vi "UHR-Fleezers Control (host) - Avogadro v2.vi"() -> ()   [LabVIEW 2014]
uses:
  <vilib>/Utility/miscctls.llb/LVPoint32TypeDef.ctl
  <vilib>/Utility/miscctls.llb/LVMinMaxIncTypeDef.ctl
  <vilib>/addons/database/Connection.llb/Conn ObjectReference.ctl
  <vilib>/sound2/lvsound2.llb/Sampling Mode.ctl
  <vilib>/sound2/lvsound2.llb/Sound Data Format.ctl
  <vilib>/Platform/TimedLoop/XDataNode/timing_clust.ctl
  <vilib>/Platform/TimedLoop/XDataNode/nitl_modes.ctl
  <vilib>/Platform/TimedLoop/XDataNode/wakeup.ctl
  uFLUX control_v2/uFLUX control_v2/Pressure Control/Pressure Control.lvclass
  uFLUX control_v2/uFLUX control_v2/TTL/TTL.lvclass
  uFLUX control_v2/uFLUX control_v2/Pressure Control/Pressure Control Config.ctl
  <vilib>/userdefined/High Color/nirio_resource_hc.ctl
  <vilib>/Analysis/baseanly.llb/Mean (DBL).vi
  <vilib>/Instr/_visa.llb/VISA Configure Serial Port (Instr).vi
  <vilib>/FPGAPlugInAG/PCIe-7852R/niLvFpga_Open_PCIe-7852R.vi
  <vilib>/FPGAPlugInAG/PCIe-7852R/niLvFpga_Reset_PCIe-7852R.vi
  <vilib>/FPGAPlugInAG/PCIe-7852R/niLvFpga_Run_PCIe-7852R.vi
  <vilib>/FPGAPlugInAG/PCIe-7852R/niLvFpga_Close_PCIe-7852R.vi
  <vilib>/Utility/error.llb/Error Cluster From Error Code.vi
  <vilib>/rvi/errors/niLvFpgaAdjustHostInterfaceError.vi
  <vilib>/rvi/interface/common/niFpgaWaitOnOcc.vi
  <vilib>/express/express analysis/Spectral/Block/exnSpectralBlock spectral measurements PSD poly.vi
  <vilib>/express/express analysis/Spectral/Block/exnSpectralBlock spectral measurements PSD WFM.vi
  <vilib>/Waveform/WDTOps.llb/WDT Append Waveforms DBL.vi
  <vilib>/Waveform/WDTOps.llb/WDT Index Channel DBL.vi
  <vilib>/sound2/lvsound2.llb/Sound Output Write (DBL Single).vi
  openfpgaref.8.6.ctl
  <vilib>/Platform/TimedLoop/XDataNode/XDataNode.xnode
  <vilib>/rvi/interface/nirviOpenFPGA/nirviOpenFPGA.xnode
  openfpgaref.initrf.ctl
  FPGA Bitfiles/UHR-FleezersInst_FPGATarget_intitializeRFsyn_v1.lvbitx
  <vilib>/rvi/interface/nirviMethod/nirviMethod.xnode
  <vilib>/rvi/interface/nirviCloseFPGA/nirviCloseFPGA.xnode
  FPGA Bitfiles/UHR-FleezersInst_FPGATarget_UHR-FleezersCont_avogadro4_switch_test.lvbitx
  <vilib>/rvi/interface/nirviReadWriteControl/nirviReadWriteControl.xnode
  <vilib>/express/express analysis/Spectral/XNode/ExpressSpectralMeasurementsBlockNode.xnode
  <vilib>/Analysis/NI_AALBase.lvlib
  <vilib>/Platform/TimedLoop/XDataNode/XDNodeRunTimeDep.lvlib
  Duncan Nall/Fluorescence simulation/Global for fluorescence simulation mean (30 samples), (power series).vi
  <vilib>/gmath/NI_Gmath.lvlib
  <vilib>/addons/database/NI_Database_API.lvlib
  <vilib>/rvi/errors/niLvFpgaMergeErrorWithErrorCode.vi
  NiFpgaLv.dll
  <vilib>/FPGAPlugInAG/PCIe-7852R/niLvFpga_ConfigureFifo_PCIe-7852R.vi
  <vilib>/FPGAPlugInAG/PCIe-7852R/niLvFpga_ReadFifo_PCIe-7852R.vi
  <vilib>/addons/database/Connection.llb/DB Tools Open Connec (Path).vi
panel:
  out "2D values (force/position/raw)":T1={"A_X"=10.819281125703213, "A_Y"=-5.499317852510465, "B_X"=12.368914072758173, "B_Y"=-10.556033598869238, "C_X"=11.443452130367886, "C_Y"=-14.04467976971868}
  out "APD rates cluster":T2={"APD 1 Rate (Hz)"=4.0, "APD 2 Rate (Hz)"=0.0, "APD 3 Rate (Hz)"=0.0, "Sigma/Mean 1"=nan, "Int Time (s)"=4.0, "Sigma 1"=0.0, "Sigma 2"=0.0, "Sigma 3"=0.0, "Sigma/Mean 2"=nan, "Sigma/Mean 3"=nan}
  out "Read offset current":string(combo)
  out "PSD Y Sum":dbl[](array[numeric])
  out "log file ref":refnum<file>
  out "AL Running":bool
  in  "AL Delay (s)":u32
  in  "Stop assembly line":bool
  in  "Cy5 Fl.  Thresh. (kHz)":dbl=24.5
  in  "Cy3 Fl.  Thresh. (kHz)":dbl=19.0
  in  "Get Fluorophore":bool
  out "Red Fluorophore":bool
  out "Green Fluorophore":bool
  in  "Numeric":dbl
  in  "stop":bool
  in  "Start assembly line":bool
  out "HP3 Flush Time (s)":dbl=90.0
  out "HP1 Flush Time (s)":dbl=60.0
  out "TTrig":cluster{dbl, dbl}(graph)
  in  "Sample Channel\nFlow":bool
  in  "Inject Pump 1":bool
  in  "Inject Pump 3":bool
  in  "Pump 1 contents":string="Bottom: DNA beads" caption="Contents"
  in  "Pump 3 contents":string="Top: ADig beads" caption="Contents"
  in  "Scripts":T3(tab)=enum."Saving"
  in  "Experiment position":bool
  in  "Get Bead 1":bool
  in  "Fixed Traps Data\nScript":bool
  in  "Dump spot flow on?":bool=TRUE caption="Flow ON?"
  in  "Daq spot flow on":bool=TRUE caption="Flow ON?"
  in  "Cap 1 Samp Flow ON":bool=TRUE
  in  "Cap 2 Samp Flow ON":bool=TRUE
  in  "Get bead 2":bool
  in  "Get bead 3":bool
  in  "Cap 2 Flow ON":bool=TRUE
  in  "Cap 1 Flow ON":bool=TRUE
  in  "Cap 2 T ON":bool=TRUE
  in  "Move Cap. 2 (ADig Top)":bool
  in  "Move Cap. 1 (DNA Bottom)":bool
  in  "Cal/Data Acq. Spot":bool
  in  "Dump Beads":bool
  in  "Cap 1 T ON":bool=TRUE
  in  "Force FB Data\nScript":bool
  in  "Cap. 2 BD T1?\n(ADig T1, DNA T2)":bool
  in  "Flow Cal":bool
  in  "Pulse Duration (0-100 ms)":dbl=10.0
  in  "Number of pulses For laminar flow":i32=1
  in  "Vent pressure":bool
  in  "Pressure Up":bool=TRUE
  in  "Pressure Down":bool=TRUE
  out "Pressure":dbl=0.010543157373989365 format="%#.2f"
  in  "Set zero pressure":bool caption="Vent pressure"
  in  "Vacuum":bool=TRUE
  in  "DAQmx Device Name":tag="Dev1"
  in  "Offset raster?":bool
  in  "MCL offset scanning range (V)":T4={"Min X"=6.0, "Max X"=9.0, "Min Y"=5.0, "Max Y"=8.0, "Scan increment"=1.0}
  in  "Multiple-MCL offset?":bool=TRUE
  in  "Active cal after cal?":bool
  in  "Fish after cal?":bool
  in  "Flow ON during cal?":bool
  in  "Offset 2 Set":dbl=3.0
  in  "Offset 1 Set":dbl
  in  "Cal @ (MHz)":dbl=14.0
  in  "W/ Offset 1":bool
  in  "Offset 1 Start (MHz)":dbl=10.0
  in  "W/ Offset 2":bool
  in  "Offset 2 Start (MHz)":dbl=10.0
  in  "Cal Stage Position":i32=3
  in  "Index":dbl=1.0 caption="Save File Index" min=1.0 step=1.0
  out "Time (s)":dbl=12.200000000000001
  in  "Channel 3 Buffer":string="NA"
  in  "Channel 2 Buffer":string="NA"
  out "Save Data Period (s)":dbl=0.001 caption="Period (s)" format="%#_6p"
  out "Save Data Rate (Hz)":dbl=1000.0 caption="Rate (Hz)" format="%#_6p"
  out "Progress":u16(slide) scale=0.0..100.0
  in  "Stop Saving":bool
  out "Saving...":bool
  in  "Save ave N":dbl=100.0 caption="Averaging Factor"
  out "Save file name":path=path "C:/Data/180326/180326_017.dat"
  in  "Save N Sets":bool
  in  "N sets to save":u32=200 caption="N Sets"
  out "Calibrating Trap...":bool
  in  "Comment (data description)":string="testing confocal setup"
  in  "Start Saving":bool
  out "Total Time (s) 2":dbl=40.0
  in  "Name":string="test name"
  in  "Title":string="testing database"
  in  "DNA Construct":string="oligo binding"
  in  "Channel 1 Buffer":string
  in  "Bead diameter":dbl=800.0
  in  "Save Event Log?":bool=TRUE
  in  "Only check fixed trap T2":bool
  in  "Flow ON after\ntether testing?":bool
  in  "Flow ON during \nfishing?":bool
  in  "Fish again after \nraster break?":bool
  in  "Furthest Delta (MHz)":dbl=15.0 step=0.25
  in  "Green ON During Raster":bool
  in  "Move to Delta 2 (MHz)":dbl=12.3
  in  "Attempt Limit":dbl=20.0 caption="Limit"
  out "Attempts":dbl=10.0
  in  "Wait Before Save (s)":u32=1
  in  "Closest Delta (MHz)":dbl=8.0 step=0.25
  in  "Stop F (pN)":dbl=3.0
  in  "Then...":string(combo)="5"
  in  "Move to Delta 1 (MHz)":dbl=10.0
  in  "Tether Alarm?":bool=TRUE
  out "Tether":bool
  in  "TA Cancel Save?":bool
  in  "TA Green Off?":bool
  in  "Raster Set Upon Tether":u32=5
  in  "Save at end (5, 6)":bool
  in  "Stop Fishing When Tether":bool=TRUE
  in  "Delay before dipping (s)":dbl=5.0
  in  "Start dipping after?":bool
  in  "Green ON after FB ON?":bool
  in  "Remove Action Offset":bool
  in  "Stage Position To Establish FB":i32=3
  in  "Trap Trig Fl.":bool
  in  "Starting \nTrap Delta (MHz)":dbl=15.25
  in  "Trap Delta Before Moving":dbl=13.0
  in  "Wait (s)":u32=1
  in  "Green ON":bool
  in  "Start dipping after?":bool=TRUE
  in  "Fixed Traps Trap Delta (MHz)":dbl=15.25 caption="Trap Delta (MHz)"
  out "TTrig Fin Thresh (nm)":dbl
  out "TTrig Sig (nm)":dbl
  out "Threshold stored (nm)":dbl
  in  "Neg. TTrig FPGA":bool=TRUE
  in  "Test ttrig":bool
  in  "Trap Trig. (FPGA)":bool=TRUE
  out "Initializing":bool
  in  "Reinitialize":bool
  out "Triggered":bool
  out "Waiting":bool
  in  "Trap Trig. Fl.":bool
  in  "Wait to get offset (n)":u32=10
  in  "Threshold (nm)":dbl=15.0
  in  "Fl. ON time (n)":i32=90
  out "max value":dbl=-0.9003514563721442
  out "min value":dbl=-1.184251119672945
  in  "Mean T1 Position\nto compare (nm)":dbl caption="Mean T1 for Comparison (nm)" format="%0.2f"
  out "mean":dbl=-1.0423012880225446 format="%0.2f"
  out "standard\ndeviation":dbl=0.2007473770965739 format="%0.2f"
  out "TTrig Sig (Int)":i64
  out "TTrig Fin Thresh (Int)":i64
  in  "FB Trig Integrate":u32=1
  in  "Green ON\nafter start\nreturn?":bool
  in  "Green delay after \nstart return (s)":dbl
  out "Dwell Time (s)":dbl
  in  "FB OFF when \nflow ON":bool
  in  "Flow ON \nduring return\nfrom dip?":bool=TRUE
  in  "Flow ON\nduring daq?":bool=TRUE
  in  "Flow ON\nduring dip?":bool=TRUE
  in  "Cancel dwell":bool
  in  "Pause dwell":bool
  in  "Dwell Duration (s)":i32=45
  in  "Green ON\nbefore dip?":bool
  in  "Cont. Repeat Dipping?":bool=TRUE
  in  "Dipping Delta (MHz)":dbl=15.0
  in  "Move trap \nbefore dip move?":bool
  in  "Save data after return?":bool
  in  "Green ON \nafter return?":bool=TRUE
  in  "Dip Trap Delta 2 (MHz)":dbl=15.0
  in  "Move trap after return?":bool
  in  "Dip Duration (s)":i32=15
  in  "Dip for Protein":bool
  in  "Dip Stage \nPosition":i32=5
  in  "Return Stage \nPosition":i32=3
  out "Dip Time (s)":i32=16
  out "Dip #":i32=5
  in  "Y change (mm)":dbl=-3.0
  in  "Profile":bool
  out "Current Position":cluster{dbl, dbl, dbl}={1.6, 0.50781, -0.0311}
  in  "Shift confocal":bool
  in  "Auto F Reset":bool
  in  "Yank when?":bool
  in  "Yank to which?":bool
  in  "Yank to SP":dbl[](array[numeric])=[-0.128, -0.158, -0.183, -0.21, -0.01, -0.0319, -0.094, -0.143]
  in  "APD to Watch":bool
  out "Duration (s)":dbl=8.399999999999977
  in  "Action":string(combo)="Yank"
  in  "Fl. Triggered...":bool
  in  "Fl. Delta Thresh. (kHz)":dbl=0.14
  out "Waiting":bool
  out "Fl. High":bool
  in  "N pts to average":u16=6
  in  "Yank Delay (s)":dbl=3.0
  in  "Yank to Trap Delta (MHz)":dbl[](array[numeric])=[16.3, 15.85, 14.85]
  in  "N Array El":u8=4 min=1 step=1
  in  "Random Choice":bool=TRUE
  in  "Force Yank":bool
  in  "Reset Force":bool
  in  "N Steps":dbl=20.0
  in  "Step Size (nm)":dbl=0.34
  in  "Save ave factor":dbl=1.0
  in  "Take Stepping Data":bool
  out "Waveform Graph":dbl[](graph) caption="APD Line Scan"
  out "Messages":string="8:21 AM\tUHR-Fleezers ready.\r"
  in  "APD Ave N":dbl=20.0
  in  "Stop All":bool=TRUE
  in  "Tab Control 6":T5(tab)
  in  "Chart APD?":bool
  in  "Pair to \nanalyze":enum16{"1-2", "2-3", "3-1"}(ring)
  in  "APD 3 Offset":dbl
  in  "APD 2 Offset":dbl
  in  "APD 1 Offset":dbl
  out "RMS (Ang)":dbl=0.5856452091881293 format="%_2g"
  in  "Bead Sep. Int. Time (s)":dbl=3.0 caption="Int. Time (s)"
  in  "Below (kHz)":dbl=1.0
  in  "Above (kHz)":dbl=2.0
  in  "Adjust Scale\nto Mean":bool
  in  "Remove Offset":bool
  in  "Offset (nm)":dbl format="%#_3g"
  out "Mean":dbl=-0.7748164735274798 caption="Mean (pN)" format="%#_3g"
  out "Force":waveform(dbl)[](graph)=[{"t0"=timestamp(907.4000000000693 s since 1904-01-01), "dt"=0.1, "Y"=[10.809672659724802, 10.828889591681625], "attributes"=variant("NI_ChannelName"=variant(string "Trap 1 X"))}, {"t0"=timestamp(907.4000000000693 s since 1904-01-01), "dt"=0.1, "Y"=[-12.364602742140338, -12.37322540337601], "attributes"=variant("NI_ChannelName"=variant(string "Trap 2 X"))}, {"t0"=timestamp(907.4000000000693 s since 1904-01-01), "dt"=0.1, "Y"=[-0.7774650412077682, -0.7721679058471924], "attributes"=variant("NI_ChannelName"=variant(string "Mean"))}]
  out "APD Chart":waveform(dbl)[](graph)=[{"t0"=timestamp(907.4000000000693 s since 1904-01-01), "dt"=0.15, "Y"=[0.0], "attributes"=variant("NI_ChannelName"=variant(string "APD 1"))}, {"t0"=timestamp(907.4000000000693 s since 1904-01-01), "dt"=0.15, "Y"=[0.0], "attributes"=variant("NI_ChannelName"=variant(string "APD 2"))}, {"t0"=timestamp(907.4000000000693 s since 1904-01-01), "dt"=0.15, "Y"=[0.0], "attributes"=variant("NI_ChannelName"=variant(string "APD 3"))}]
  in  "Calibration":u16(ring)=2 items=["None", "Position", "Force"]
  out "T1 X":dbl=10.819281125703213 caption="T1 X (pN)" format="%0.2f"
  out "T2 X":dbl=-12.368914072758173 caption="T2 X (pN)" format="%0.2f"
  out "Bead Separation":waveform(dbl)[](graph)
  out "Bead Mean (nm)":dbl=3063.2633875359443 caption="Mean (nm)" format="%0.2f"
  out "Difference":dbl=23.188195198461386 caption="Difference (pN)" format="%.2g"
  out "Trap Positions":waveform(dbl)[](graph)=[{"t0"=timestamp(907.4000000000693 s since 1904-01-01), "dt"=0.01, "Y"=[2029.9999999999682, 2029.9999999999682, 2029.9999999999682, 2029.9999999999682, 2029.9999999999682, 2029.9999999999682, 2029.9999999999682, 2029.9999999999682, 2029.9999999999682, 2029.9999999999682, 2029.9999999999682, 2029.9999999999682, 2029.9999999999682, 2029.9999999999682, 2029.9999999999682, 2029.9999999999682, 2029.9999999999682, 2029.9999999999682, 2029.9999999999682, 2029.9999999999682], "attributes"=variant("NI_ChannelName"=variant(string "Trap 1 X"))}, {"t0"=timestamp(907.4000000000693 s since 1904-01-01), "dt"=0.01, "Y"=[6090.0, 6090.0, 6090.0, 6090.0, 6090.0, 6090.0, 6090.0, 6090.0, 6090.0, 6090.0, 6090.0, 6090.0, 6090.0, 6090.0, 6090.0, 6090.0, 6090.0, 6090.0, 6090.0, 6090.0], "attributes"=variant("NI_ChannelName"=variant(string "Trap 2 X"))}, {"t0"=timestamp(907.4000000000693 s since 1904-01-01), "dt"=0.01, "Y"=[3856.3118985290066, 3856.3118985290066, 3856.3118985290066, 3856.3118985290066, 3856.3118985290066, 3856.3118985290066, 3856.3118985290066, 3856.3118985290066, 3856.3118985290066, 3856.3118985290066, 3856.3118985290066, 3856.3118985290066, 3856.3118985290066, 3856.3118985290066, 3856.3118985290066, 3856.3118985290066, 3856.3118985290066, 3856.3118985290066, 3856.3118985290066, 3856.3118985290066], "attributes"=variant("NI_ChannelName"=variant(string "Trap 3 X"))}, {"t0"=timestamp(907.4000000000693 s since 1904-01-01), "dt"=0.01, "Y"=[-2.7867843867294573, -2.7867843867294573, -2.7867843867294573, -2.7867843867294573, -2.7867843867294573, -2.7867843867294573, -2.7867843867294573, -2.7867843867294573, -2.7867843867294573, -2.7867843867294573, -2.7867843867294573, -2.7867843867294573, -2.7867843867294573, -2.7867843867294573, -2.7867843867294573, -2.7867843867294573, -2.7867843867294573, -2.7867843867294573, -2.7867843867294573, -2.7867843867294573], "attributes"=variant("NI_ChannelName"=variant(string "Trap 3 Y"))}]
  in  "Plot Trap Positions":u16(ring)=1 items=["Relative to Base", "Absolute Positions"]
  out "Mean Trap Positions (nm)":T6={"T1 X"=2029.9999999999682, "T2 X"=6090.0, "T3 X"=3856.3118985290066, "T3 Y"=-2.7867843867294573} {"T3 Y" format="%#_6f"; "T3 X" format="%#_6f"; "T2 X" format="%#_6f"; "T1 X" format="%#_6f"}
  out "Trap RMS (ang)":T6
  in  "FB Trap Pos Offset":dbl=-9.744913000168507 caption="Offset (nm)" format="%.1f"
  in  "Rem fb disp offset":bool caption="Rem. Offset"
  in  "Negate Axis":T7
  in  "Trap Pos. Disp. Downsample":dbl=1000.0 caption="Trap Downsample"
  out "Current deltaF (MHz)":dbl=20.00000000000024
  out "Confocal Y 2 (V)":dbl=6.809280068361465
  out "Confocal X 2 (V)":dbl=0.7223435163426621
  out "Confocal Y 1 (V)":dbl=0.7905362102114931
  out "Confocal X 1 (V)":dbl=4.726554155095066
  in  "Set High F Confocal Spot (X-Y)":bool
  in  "Take Detection Laser\nImage":bool
  out "APD 2":T8(plugin-control) caption="APD 2 (Cy5)"
  in  "Flip Green Filter":bool
  in  "Set X Only":bool
  in  "Set Y Only":bool
  out "APD 1":T8(plugin-control) caption="APD 1 (Cy3)"
  out "Detection Laser Y":T8(plugin-control)
  out "Pointer Y (V)":dbl=1.4785302285836357 format="%_3g"
  out "Pointer X (V)":dbl=-0.03375347148045271 format="%_3g"
  in  "Set Confocal Spot (X-Y)":bool
  out "Detection Laser X":T8(plugin-control)
  out "APD 3":T8(plugin-control) caption="APD 3 (Cy2)"
  in  "Display Saved Data":string(combo)
  out "Saved trap pos":dbl[](graph)
  out "Saved APD":dbl[][](graph) caption="Most Recent Time Trace"
  out "Trap Delta Graph":dbl[](graph)=[-888.5232584479509, -892.5692760325692, -888.5232584479509, -892.5692760325692, -891.2360697801105, -894.3600396459187, -891.3530490659778, -892.9679669132674, -887.2494984625082, -888.47771676923, -888.6329185051081, -889.7156495337531, -889.1930112791088, -888.4045039038392, -888.084843029651, -889.8875525920621, inf, -891.5676283442608, -894.5094286061385, -891.5983606475702, -893.1878191776686, -891.3325610057909, -893.6093263444927, -896.2367307427394, -892.2217144646074, -894.9535690358598, -887.956521414997, -890.7739120767728, -893.0602682588451, -895.1640366432557, -892.7910234320525, -893.1772797409612, -888.0283778908597, -892.2886839318544, -892.7242287695717, -891.8394715865525, -892.6628927156271, -891.8793537272368, -893.5686832780566, -894.0582980429208, -895.6882905161083, -895.890842543693, -894.3130596329747, -892.7737317546289, -894.0385259825343, -894.1252619934476, -896.980108376255, -896.6022964762888, -892.1152046899178, -898.8619004796719, -892.4324256979044, -895.0928134296864, -903.0784997671863, -902.9498086361546, -904.0153255210525, -901.4622120705908, -901.9721056496455, -904.6740753274289, -901.8902972234864, -903.3842915230061, -900.3250329838766, -898.9820691503892, -901.1294317229076, -905.01552371458, -904.6763511570998, -903.2505279614516, -902.3941327474286, -903.6395081819228, -906.0026468208371, -905.0720047317454, -905.1166548814244, -904.0489605368157, -902.8812750877614, -905.7991217269264, -903.6875202921092, -907.4124074209194, -904.7140083836757, -904.8350869111428, -902.6570916377068, -905.9840520542539, -904.721341571344, -901.3835199864006, -900.6377520988308, -903.5252999725608, -902.2998714272662, -906.1753928616326, -902.4085864251283, -907.4909598319209, -903.7987350858766, -908.5563805038573, -906.7982006835309, -904.532239502093, -904.7744981129244, -902.8763684599026, -905.1603694736959, -906.5327087472069, -904.6649386135277, -904.1928399602957, -905.4849901818643, -904.4683250224571, -899.6358046887099, -904.5973964541627, -906.9313496550249, -904.7524096784455, -907.6988597728841, -908.916844755332, -910.1663235260221, -908.8075013013076, -905.8028727577857, -905.8045997029394, -906.9113332645784, -908.3503633772207, -907.4784268045696, -905.5720759063224, -906.3984489455179, -907.3393783713009, -907.8177849485846, -906.9360070315706, -907.6999060274848, -908.2881615331507, -907.077718922088, -906.8617653154515, -904.9424603989628, -907.0937893053306, -907.5590092972907, -908.1623052224686, -904.2223991103392, -906.3563736167625, -905.0225392735301, -905.295681302322, -906.4651827134403, -903.2439008203055, -905.7693911282695, -905.7682551298649, -906.7772876249264, -903.4235808464164, -909.1265231000943, -903.4976056084442, -905.1013467234716, -902.6253676788865, -902.5559161171359, -905.9900448685412, -908.3060573669163, -908.271057609043, -908.6249955191133, -908.4649190879954, -908.0436156500946, -910.473173178445, -909.1062905650151, -910.7079613122369, -907.4250280029873, -905.6076025935581, -898.8088905447858, -903.402409375125, -901.7095176037255, -900.6553838720265, -902.79475305087, -904.3955242157135, -903.1247032365154, -906.0436268803969, -902.8275123571893, -902.796487377057, -901.0943487511367, -905.2411242572371, -900.8483242955845, -901.1701267046437, -901.2359067441666, -906.3090266542558, -903.203719534853, -908.5826070839084, -904.3524089878192, -905.4734019775005, -902.9956995180391, -902.6158584118066, -899.1327939065986, -902.2376916026697, -905.103004143929, -903.1277607411912, -903.6282471067552, -907.0682312311483, -906.2221787991994, -902.6411693211257, -902.094737311153, -904.7468905996429, -902.1336079862131, -901.5952820446182, -900.9632702019098, -897.7125842088453, -902.8760170565547, -904.4362988516959, -902.4817145305642, -901.7625765951907, -898.5102238195077, -903.537745400934, -896.3444926998609, -901.259842380422, -897.5436321469942, -898.952050106539, -900.6692781312959, -901.1593068029997, -898.4323281846864, -903.0845906105824, -995.9731275252025, -995.9947934967686, -995.9799414488389, -996.0073955110902, -995.9579761572559, -995.9711910119959, -995.9774583854778, -995.9575528392079, -995.9561349901087, -995.9542751868667, -995.9774991705708, -995.9616897494452, -995.9757905332817, -995.9908471851622, -995.9739909085556, -995.9718114419275, -995.9959525512286, -995.9844131558621, -995.9904908641547, -995.9889391909255, -996.0028641968001, -996.0013951079109, -995.9810763138194, -995.9810382746236, -995.9911722439219, -995.9859667223, -995.9851436026411, -995.9939001721541, -995.9865114348904, -995.9814983567767, -995.9952810967052, -995.9903559276554, -995.9866410688073, -995.9880059400593, -995.9789809636295, -995.9963936860495, -995.9578036566736, -995.9625570794387, -995.9999889501587, -995.9968505444012, -996.0080660533258, -995.9921435696897, -995.9758019434594, -995.9999828587006, -995.9546174673769, -995.9798304990454, -995.9889307200046, -995.9725720635597, -995.9903044730327, -995.9637012167495, -991.7799569235185, -991.8322696856321, -991.782331348857, -991.8032950721445, -991.7590045489951, -991.7823921026202, -991.8106735781785, -991.8241562576231, -991.8538929551651, -991.7318190532487, -991.7036942962213, -991.6413248254112, -991.5087149122355, -991.488745354497, -991.6037009177753, -991.5953354830326, -991.7547211463634, -991.5376992417932, -991.440699211259, -991.5124866576461, -991.4991944712829, -991.7223810385476, -991.726748717816, -991.8932683475532, -991.7763611344299, -991.7850735913107, -991.8024211296206, -991.8224857741852, -991.9723950863772, -991.7320104833734, -991.7934342846875, -991.7851145268105, -991.7432232831488, -991.7405675679238, -991.909709033087, -991.6940380436636, -991.7324235075157, -991.5854261711766, -991.5851972637411, -991.7038504715401, -991.7874392998519, -991.6887154536307, -991.7279006008021, -991.6715868379915, -991.6784740216681, -991.7032274760013, -991.7644533951507, -991.759143130872, -991.5925750049673, -991.7640627193787, -994.953208627312, -995.0063050032368, -994.9662702686564, -995.026749751938, -994.925346906377, -994.9524396568559, -994.9762699468374, -994.8771378794718, -995.0064143618201, -994.954850544249, -994.9462016870275, -994.9109430986919, -994.9112665819885, -994.9771341378473, -995.0189767272732, -994.9862664173124, -994.9857435262275, -995.0083929437715, -994.949812407076, -995.010867385572, -995.000315449437, -994.9751627983078, -995.0242807778759, -995.0256740318546, -994.9955484130642, -995.0195738481034, -995.0972681265357, -995.0731533889957, -994.9480975319966, -994.9426357529683, -994.9859546616735, -995.0406814051694, -994.9585320470287, -995.0613507745657, -994.9820163627555, -995.0726183216902, -994.9744204423059, -995.056348643795, -994.958647093612, -994.997406895005, -995.0347073088487, -995.0001414461567, -995.0656194283056, -995.0250982611306, -995.0367867247915, -995.0677311523086, -995.0718547788274, -995.0152755454492, -994.9939420977498, -994.9995846174152, -996.2112978835139, -996.1937551973788, -996.3253378148002, -996.2486992120994, -996.2797935177368, -996.1528502860037, -996.2307760687036, -996.1697066124034, -996.2001992217083, -996.2381980836853, -996.2607883274868, -996.1772511301369, -996.2931686016091, -996.2067304537395, -996.2985477880102, -996.3293824680932, -996.2782599101029, -996.3372206906879, -996.3241174705418, -996.3338106632746, -996.3562091215554, -996.3215684207953, -996.322015361473, -996.3579748510183, -996.3984694095925, -996.4247913247564, -996.3431055963356, -996.4001770726845, -996.2744724635177, -996.3628817626523, -996.3689572110452, -996.3762233750731, -996.3733535425563, -996.3960143128006, -996.3482281752404, -996.4428932001993, -996.3941617900255, -996.3710775427589, -996.3744761888029, -996.3870099915403, -996.3942686053178, -996.3005753926991, -996.371086148536, -996.2713205328728, -996.372847637309, -996.3758150101294, -996.3526029356217, -996.3049625746025, -996.242517365732, -996.31050454869, -997.6111781026066, -998.6501705777573, -998.1132395809478, -994.5425674374171, -998.2660703252495, -994.7083172779076, -998.798975472464, -997.6122000704445, -995.8364679745928, -999.4985112855938, -993.0656663235804, -996.5081392146012, -990.1291317184978, -993.3763588849524, -986.8975878683968, -990.2360604230744, -983.6497631530901, -986.8520561070509, -980.3603561743366, -983.5158483768964, -976.8208114210456, -979.9834326724958, -973.1431995631328, -976.3015508745984, -969.3158794424162, -972.3865185335599, -965.3801624532043, -968.1859985463634, -961.288207771936, -964.1268282652409, -956.9679865110638, -959.8200925928586, -952.694063463674, -955.462798759143, -947.9472723622684, -950.5960046016298, -943.2287940912547, -945.7419861823664, -938.1651014048794, -940.5427534305672, -932.8483329282681, -935.1767245131487, -927.5533890759807, -929.7205795758646, -921.7491056131485, -923.8880060146066, -915.7798826664175, -917.6504396174314, -909.3477658222437, -911.1010619947447, -902.9750174360652, -904.542794009215, -896.1621635262263, -897.4763693613477, -889.0871358962386, -890.4038112090375, -881.8471528446989, -883.1100643850314, -874.469691051514, -875.4468076792791, -865.454075287279, -864.2719956982637, -859.7513847939963, -858.5141975792885, -862.1280808539414, -860.8821364963351, -869.3191212367556, -868.0137786842088, -876.1838475466739, -874.4200872092661, -882.7870665996597, -880.9796913538194, -889.275397673794, -887.330353880735, -895.3904446874203, -893.1797717248119, -901.3273277635526, -898.9207711668314, -906.7897146720752, -904.3678364059051, -912.1524755193886, -909.6985355057814, -917.2987633922403, -914.661370647068, -922.2142329673416, -919.6044536379841, -927.1223416219191, -924.3154747273229, -931.5638309544656, -928.7549540980581, -935.8266822463565, -932.9774203262577, -940.1163171386979, -937.1564299426345, -944.0009520995081, -941.0386104590079, -947.8786276127548, -944.8118311537874, -951.6648506899492, -948.4458673337813, -955.3028715958089, -951.9160121960595, -958.5071565951321, -955.2223572371822, -961.8793841757006, -958.59866436005, -965.014881911241, -961.7404216546402, -968.1657693012967, -964.7561380615289, -971.1693559247788, -967.66615131466, -974.0841481997004, -970.5363911806962, -977.0088587087284, -973.5505650167443, -979.877831187543, -976.2553013966917, -982.6585054904217, -978.9230705650871, -988.9292563673525, -992.7300236601677, -999.6075741350014, -996.8134832896676, -998.2574907173475, -994.6404336239739, -998.8693447346323, -997.6540718154065, -995.9261472571197, -999.4658744090393, -993.140444883913, -996.6010456968861, -990.1133827575668, -993.4405787333353, -986.9598171440912, -990.3926389646558, -983.7163049255614, -987.1192322505331, -980.4391572155519, -983.7920093505809, -977.0000419842945, -980.2490670266625, -973.3863615483951, -976.5955827608695, -969.6973709355898, -972.7700169554655, -965.8333414432882, -968.717614754114, -961.7186454223647, -964.5704781273735, -957.4294357216122, -960.1950234098331, -953.118095314423, -955.7834990905794, -948.5368059535203, -951.0671218694561, -943.655724555927, -946.1558455361264, -938.4991902731454, -940.9420946361488, -933.1755978246201, -935.4919219237618, -927.9830415993483, -930.0736968419387, -922.3289608890236, -924.3131242097106, -916.0762607591969, -918.0280788611626, -909.9778363244104, -911.649487787704, -903.3981843187685, -905.1266746062611, -896.7219645395735, -898.0799703834773, -889.6712193743151, -890.998358986295, -882.4572023550118, -883.666561319229, -874.9235768085673, -875.9311434212259, -865.8516706595301, -864.7516300642255, -860.2323973486937, -858.913243482376, -862.5308481449747, -861.1476813387144, -869.5735125168903, -868.0792658929731, -876.7972647810657, -874.9041687732488, -883.3291770015549, -881.3509461882468, -889.7371441249652, -887.6779536606336, -895.7113582832062, -893.7279693095934, -901.745228423516, -899.5764408890209, -907.1077290683097, -904.8979939291221, -912.5465767880314, -910.0961331374428, -917.7025950009729, -915.0994152690791, -922.6196551978846, -919.953705517024, -927.3159321943886, -924.6073757165359, -931.8266946984295, -928.975770151058, -936.1252531542432, -933.2685428588757, -940.2856308615628, -937.3674132176293, -944.3130518907556, -941.23216916824, -948.1478220469435, -945.0406175847211, -951.9316708269935, -948.7768773475736, -955.5222855383181, -952.2615618852888, -958.7063401858923, -955.4993735387097, -962.118828737317, -958.6174131606767, -965.2509805388854, -961.8371585431678, -968.2994221730896, -964.8333111974634, -971.1577258358393, -967.663343918679, -974.1440521791928, -970.6008463569397, -977.0498586244403, -973.4959773098299, -979.9642181209001, -976.2956827150274, -982.8034163990687, -979.0438654247, -989.0302813305561, -992.8074830460873, -999.6867303598647, -996.8003818690731, -998.2222715269954, -994.6763354148452, -998.8653021701639, -997.5563362912735, -996.0284279346961, -999.5870695225167, -993.1519142195602, -996.6060728842358, -990.1174730499197, -993.5857415877254, -987.0910284137999, -990.2921782513013, -983.7785143765741, -987.0264184618154, -980.4130118787507, -983.7759210697814, -977.0845342115672, -980.3218830432852, -973.4286467229713, -976.5190127936739, -969.6570345107202, -972.7859589548525, -965.8773115977747, -968.6529655316681, -961.6957563203287, -964.5280495626448, -957.3652767798567, -960.3475350683439, -953.0753647556021, -955.750112313046, -948.3348870284717, -951.0171373133071, -943.4279935340646, -945.9140985178674, -938.397838475491, -940.8445346761237, -933.0238204512043, -935.3254453444897, -927.6182701426706, -929.8930904129547, -921.8983600766587, -923.9432748713689, -915.8650775821461, -917.7448231164681, -909.7257861962398, -911.3823697188463, -903.1126439867867, -904.7534693144698, -896.4502076962153, -897.7657602249619, -889.2593239112193, -890.5658695080256, -882.054360043745, -883.2477540699429, -874.3140539878395, -875.7478872787269, -865.5915266601887, -864.4495418254273, -859.8801745225182, -858.5746091664978, -862.1925570708781, -860.7281946496214, -869.2051969990498, -867.834930596101, -876.2035355754451, -874.4899760743901, -882.9142214264612, -881.0927068672418, -889.3736200668009, -887.4378022795772, -895.5858920490627, -893.3849228574954, -901.3833475815791, -899.1978433230543, -906.9496100927745, -904.5187981460385, -912.5319221876889, -909.88303070658, -917.3979210554799, -914.9830435026779, -922.5862039018602, -919.8172944660273, -927.2782177235295, -924.5429129426448, -931.9461429835183, -928.9847105584622, -936.1972266600742, -933.3410737986778, -940.3694802092377, -937.366305997396, -944.3522035235574, -941.3383594909956, -948.0835620396683, -945.1479153419532, -951.9248130005308, -948.8246428773964, -955.531763074252, -952.3209221454727, -958.7721964085622, -955.5009091628581, -962.0646901715327, -958.7289187958313, -965.3640587535992, -961.9159103851334, -968.3373256767827, -964.9561269852857, -971.2942575840243, -967.7041270037753, -974.1526601015667, -970.6460602590505, -977.113347645386, -973.4515060017384, -979.9239965773868, -976.2624004022937, -982.7360302056713, -979.0079750992309, -989.0632796629043, -992.7419233910186, -999.7296053168147, -996.6964181547246, -998.1176958311307, -994.563651016455, -998.8668733961422, -997.5003438963286, -996.0976671018061, -999.7166146221543, -993.290542495035, -996.7276000999645, -990.2179182953878, -993.5605360101617, -987.0577730298237, -990.3240629547709, -983.8023995217818, -987.0615140168948, -980.3801496705046, -983.7640504739675, -976.8973128959778, -980.2722220505857, -973.4234872448333, -976.5622609736802, -969.6760371817909, -972.7068942184551, -965.8083941153045, -968.6745661891828, -961.6007309295283, -964.4179460940986, -957.4527634319311, -960.239653974053, -953.0110530312822, -955.5890786589771, -948.1173604850292, -950.740042489063, -943.5123151790476, -945.9435104278773, -938.4166319815049, -940.762014073799, -932.9091811916933, -935.2077556807508, -927.5241999947593, -929.9074695009031, -921.8935957056483, -924.0135138782935, -915.7746688993757, -917.6695728136365, -909.5236394963231, -911.4390143561868, -903.1932561608546, -904.9979957913392, -896.444458812005, -897.8580927284547, -889.505080904145, -890.7480409840291, -882.2302645233358, -883.4789624280784, -874.748292103427, -875.7592735898525, -865.8120476395416, -864.5456884139712, -860.1878623519933, -858.7553964651706, -862.552548547771, -860.9467991449728, -869.462995797755, -868.0963017954391, -876.516901168895, -874.8337297284752, -883.0804934224079, -881.372403025638, -889.5360806885383, -887.7076507114143, -895.8276910232871, -893.674292186658, -901.6674730497962, -899.360099729146, -907.2372814725941, -904.8098086849814, -912.4886771042866, -910.224274881235, -917.6950105255391, -915.2186584611045, -922.65332222082, -920.1488459340835, -927.4113840739792, -924.6969728452941, -931.7496901628438, -928.9751614322277, -936.0454679639051, -933.2085739613613, -940.0997318881173, -937.3430350535073, -944.2791501626734, -941.2153117356074, -948.0266635561647, -945.0482981302384, -951.8889647600872, -948.7771729550977, -955.621601754925, -952.299763208116, -958.8499718950761, -955.5652081125545, -962.2315874680626, -958.7546921437361, -965.3655394220123, -961.8127305917978, -968.4028325539102, -964.883704355887, -971.3711121833567, -967.6594525661494, -974.1068526274667, -970.5044938023038, -977.0213921227369, -973.4779017989849, -979.9249680098264, -976.3559405421092, -982.7844124366211, -978.9344343196808, -988.9330597420385, -992.7650840272654, -999.5323730503997, -996.8077162936543, -998.2766139315409, -994.7421347284735, -998.6120446337391, -997.6571138573318, -995.8978627223014, -999.4768021722275, -993.0974429926364, -996.5728853284836, -990.1150790319998, -993.47613336206, -986.9873610236682, -990.3464407695783, -983.7746150577887, -987.0197433360836, -980.4463359171959, -983.7074442972753, -976.8848107123322, -980.1019951184717, -973.3875656717355, -976.4486949690781, -969.6377688865805, -972.5255833059327, -965.6639665940247, -968.3856190427668, -961.537502744116, -964.426208557571, -957.3190100576276, -960.1694050524156, -952.8888275781692, -955.5301168016003, -948.2079730912064, -950.8673655091361, -943.3940770256804, -945.8800833100477, -938.3048191363632, -940.8060055625947, -932.884388199449, -935.3114049150872, -927.5529488330285, -929.8463861981036, -921.8064305171301, -923.9044874029241, -915.8489310144159, -917.6690537399954, -909.4848484502572, -911.4637658745414, -903.1507476983879, -904.6318698993455, -896.4118184612389, -897.767856592749, -889.2639716736585, -890.6367547289892, -882.0154690219315, -883.2822077806632, -874.574955784321, -875.7205319287832, -865.6102510120536, -864.491375343262, -859.9876051684632, -858.7445470568691, -862.4860091548653, -860.9612794931854, -869.5565754853478, -868.1020411824575, -876.4219675470185, -874.7148051870117, -882.9877640965515, -881.1999834517028, -889.3561165270985, -887.4739360971662, -895.5035081419273, -893.4914764447149, -901.4595937132399, -899.2781966604825, -907.015549689122, -904.6314220206696, -912.4108168053854, -910.0744349460792, -917.4840944748448, -915.0874436777594, -922.521224692011, -919.8859827199594, -927.362867769948, -924.4918828309428, -931.7744559913781, -928.9595819450724, -936.0580550956147, -933.0688605945388, -940.1774890203687, -937.2027529560191, -944.227606817487, -941.1532406458982, -948.0273859386616, -944.878326333207, -951.7208307720621, -948.4757352237675, -955.1220195085625, -951.9809042608267, -958.4905267288959, -955.2500809089925, -961.7930222923551, -958.5173563138069, -965.0417246034585, -961.6757824489187, -968.1724441735323, -964.7175541476772, -971.05701232498, -967.4657126153661, -973.9426632227542, -970.5053965698489, -976.9297813792382, -973.447605058308, -979.8831926821504, -976.3663165360704, -982.7442240638657, -978.99574180125, -997.6671903473907, -998.5760314208355, -997.9516500145037, -994.4959609067137, -998.1180328951405, -994.4963761276149, -999.0367558803209, -997.3963581243561, -996.1313498027648, -999.6509284685517, -993.2476265338728, -996.6261191100375, -990.2163555472052, -993.6377834560917, -986.9826987043261, -990.3435021523064, -983.6989009483468, -987.065207030998, -980.4873967035883, -983.8501489167329, -977.0402563689786, -980.233503620002, -973.4916622348173, -976.5984301574226, -969.6654390563563, -972.8059820216795, -965.8285697013944, -968.7774280392505, -961.7948036961943, -964.771263632515, -957.6446194423179, -960.2559145795376, -953.2806674233161, -955.8760935997916, -948.54248821092, -951.0523167372176, -943.6536107573211, -946.154592659961, -938.6113141955302, -940.9831771116214, -933.3167236217023, -935.5776990990353, -928.0271244205314, -930.183935303563, -922.2916962785912, -924.3459289137081, -916.2860007466597, -918.1664889947197, -909.8497695691458, -911.7753032635983, -903.548567624357, -905.2932174878824, -896.8516954486377, -898.3604687318657, -889.8029940287497, -891.0753442923433, -882.5567094578073, -883.9320176897954, -875.1322432604356, -876.347245297492, -866.356522981866, -865.1613852602786, -860.5581773979284, -859.3362004046021, -862.8172767735359, -861.4407178647552, -870.0166596419949, -868.6207280228828, -877.022954852655, -875.3840384295854, -883.5003990926034, -881.7348007383616, -890.0054501119057, -887.975262218929, -896.2833534372712, -894.0637387634433, -901.9493279276685, -899.7358135115755, -907.3900338637923, -905.1134735344694, -912.7055046488222, -910.405638265046, -917.8539036850043, -915.4315810633962, -922.8455175803629, -920.2323720043569, -927.4989985157035, -924.8684751187857, -932.1266944079562, -929.2740233164868, -936.4812920772602, -933.5363668347945, -940.6170247747814, -937.5707766526339, -944.6299684608994, -941.4675713586093, -948.4900744670686, -945.0764607975079, -952.091304849977, -948.8389836878505, -955.6826120160013, -952.2517609514507, -958.9061636326542, -955.61582530533, -962.2933262575189, -958.8619644990595, -965.4737403450554, -961.9394859431768, -968.3969401862769, -964.9495657119869, -971.3075667710355, -967.7876663887891, -974.1753725044973, -970.6284814537266, -977.1485207835503, -973.6090669196428, -980.0448947307877, -976.4625663304623, -982.7987827880506, -979.0658056243974, -989.0522232113399, -992.9505392489727, -999.7732028236778, -996.6060408148123, -998.003049446761, -994.4747357231681, -999.1138067840329, -997.413501383643, -996.1925152703925, -999.7574621316726, -993.2935603583037, -996.7546868238296, -990.3473853840369, -993.6684724825818, -987.2544258492771, -990.5837688458523, -984.1323177937302, -987.4387812517334, -980.8356652512057, -984.0801527411513, -977.299221835885, -980.5710882463964, -973.6564886061951, -976.8234328630306, -969.990292900573, -973.192139113672, -966.2740766194793, -969.0384481494275, -962.0641489828577, -964.9665798905653, -957.7542794878191, -960.7794597867369, -953.5538848479355, -956.2363798572223, -948.881628967677, -951.6381049278934, -944.2223860549257, -946.6390093119244, -939.1738104998703, -941.5558929637818, -933.6559707922488, -936.0933943563887, -928.3606579860943, -930.5440622672404, -922.6713546692463, -924.7102025635231, -916.706282808349, -918.729793286926, -910.5970853212448, -912.2902532186145, -904.0064083165826, -905.8251617706665, -897.2522207957545, -898.7595547706633, -890.4151397675878, -891.8340144153135, -883.0088352725761, -884.2440250218624, -875.4523512751875, -876.5870350761506, -866.722900190066, -865.598807666167, -861.0298111677093, -859.6408607896747, -863.3722874419482, -861.9693845505171, -870.2077565854879, -868.9519885512282, -877.3068649206807, -875.6654579156084, -884.0545512517874, -882.3195781577906, -890.3633623354108, -888.420470363978, -896.5612197149121, -894.4909081555179, -902.4413454166888, -900.0540944124023, -907.9933421427804, -905.5533510737896, -913.2961195205089, -910.798891059092, -918.3376242468175, -915.7144585522101, -923.3310772760206, -920.6248486972427, -928.0156889617328, -925.2900227186365, -932.5786905893792, -929.5017358053665, -936.7981105923509, -933.8409686495479, -940.7866940957456, -937.8473225215994, -944.7447257700414, -941.6827698039306, -948.5344760398939, -945.5692718499395, -952.3228283399649, -949.0768543808299, -955.8906090518758, -952.5477800398148, -959.1093032812287, -955.8404980821315, -962.2835091611887, -958.9006517180251, -965.5651751742698, -962.1099669579489, -968.477936119235, -965.036968278675, -971.5680857178577, -967.8709178832969, -974.263381648514, -970.789866878682, -977.2670813465593, -973.6772334040188, -980.1107228282226, -976.5200806403018, -982.8410395673482, -978.9457087153087, -989.022990902451, -992.7517732550095, -999.7128352722284, -996.5883633756857, -998.0907479951065, -994.4452874847448, -999.0556324922218, -997.3505950489098, -996.267005516962, -999.7298615733853, -993.3807450006416, -996.8008102480571, -990.3793271502418, -993.8148911844874, -987.2834263085906, -990.6710690730933, -984.0930350916406, -987.3649983266232, -980.9793976428164, -984.1922583842606, -977.4594452146994, -980.5677857766195, -973.9214693383956, -976.8932769469757, -970.042790284403, -973.1031003558255, -966.3068151376328, -969.1373798261375, -962.1535248103255, -964.998673207585, -957.8225205016743, -960.5749370368985, -953.4077997566592, -956.1942262679022, -948.787821554979, -951.4198759913779, -943.893038702885, -946.5262703629378, -938.931604510175, -941.5376401381773, -933.6400600489787, -936.1427887584541, -928.3121353275174, -930.6108912567533, -922.526252732061, -924.7137706301637, -916.6106289101572, -918.4596285100761, -910.293934849703, -912.1352724269791, -903.7686367332117, -905.5286281781064, -897.1166203505263, -898.5026012144617, -890.0803281554272, -891.3510455990554, -882.8581760124307, -883.9133033997769, -875.1026794421259, -876.2046971510945, -866.3612894515381, -865.0810151089181, -860.6220120624448, -859.291084956787, -863.0995894519447, -861.7824098589444, -870.0117913766908, -868.5974335161973, -877.1214811378441, -875.3935898247755, -883.7979023128855, -881.9005635892154, -890.1869870393166, -888.151838460918, -896.2928254041908, -894.1940662761117, -902.1047654854683, -899.9583687914019, -907.6206179035462, -905.0751704623017, -912.9398398268313, -910.4812853675267, -918.0402673641092, -915.4011405533893, -922.9591463988063, -920.273654496209, -927.5792590247893, -924.8643466623416, -932.0164685213504, -929.265842072733, -936.462036219973, -933.6311228130407, -940.6979460516304, -937.729937355175, -944.6227133824214, -941.6000082604414, -948.4622787115622, -945.3059596144549, -952.1268075497082, -948.8149145256011, -955.6630732335816, -952.2493317094359, -958.897637411721, -955.6183037655783, -962.213021637056, -958.8154795076589, -965.5510968381477, -961.906891705491, -968.4774260786908, -964.8982621511877, -971.2909817013888, -967.656417369185, -974.1300889878667, -970.6664444734733, -977.010948530904, -973.5179495911725, -980.0027358370071, -976.4033919798485, -982.7470482004028, -978.9891822121936, -988.9548164989819, -992.7441270055251, -999.5505472233044, -996.8184610673397, -998.1843703770774, -994.6000913636517, -998.9046682548742, -997.4444620953154, -996.042857230771, -999.5797712831072, -993.17840407329, -996.6330995481339, -990.3387676979291, -993.779211652276, -987.2246827000145, -990.5894493459418, -983.9815491865984, -987.2761104336523, -980.7223641057308, -983.9873121541896, -977.1887946094621, -980.4937838543492, -973.6154860396728, -976.7996706990334, -969.9109955596687, -973.011534509893, -966.0097042189609, -968.8717329331112, -961.916536310724, -964.7476272784206, -957.7404522001061, -960.5850872489409, -953.5047646007661, -955.9400416147482, -948.7394033558267, -951.2897969594333, -943.9227841364072, -946.3652921258035, -938.8236497564021, -941.1091778244945, -933.4545131461182, -935.8258648474475, -928.1244454418102, -930.2882476471286, -922.4692464566542, -924.5587168732927, -916.5362035336739, -918.4495505756113, -910.3149132165008, -912.0886187230444, -903.9345651064277, -905.5747631973609, -897.2214095688723, -898.7312355051845, -890.1279815932767, -891.5773706059999, -883.0037556693123, -884.2585275000274, -875.4913714414179, -876.7551805632584, -866.6182001779898, -865.4993556051013, -860.9517791529561, -859.7513324850452, -863.4401528541639, -861.8730930534639, -870.3791505894387, -868.9954265751203, -877.3711680924616, -875.7504244902339, -883.9391278257617, -882.1974983850014, -890.283714175478, -888.3804535809468, -896.5019270892753, -894.3591344428978, -902.3654086627184, -899.9512212758918, -907.705002186015, -905.3107824949211, -913.1311706731049, -910.7654497141448, -918.2925885561563, -915.6668984238822, -923.204245149117, -920.5047997567608, -927.9121605789023, -925.1670591589591, -932.4493195594969, -929.4598946793039, -936.6438732282895, -933.778527318037, -940.727344442259, -937.8947948331088, -944.884747948945, -941.7565184157047, -948.60707633128, -945.5316275329087, -952.2993267180145, -949.1344927424689, -955.8695820134535, -952.6537312666505, -959.0044641042387, -955.8268137279019, -962.2598230159929, -959.0152273982003, -965.4827869624651, -962.1509544075989, -968.5487333763449, -965.0870585183557, -971.493027698245, -967.9064686372267, -974.3029887350867, -970.8561574355972, -977.2850868211453, -973.7827233113985, -980.1110728438589, -976.4525215807926, -982.9805727235989, -979.1773916703241, -989.1462538851665, -992.9415978952602, -999.836987978173, -996.5702417287166, -997.8893490857054, -994.3995301418554, -999.2126617348276, -997.3953539283848, -996.2994495715993, -999.7440286601168, -993.3982077390465, -996.7784807020435, -990.4714306347742, -993.95007475287, -987.3543477796338, -990.7712515149688, -984.1702673949958, -987.4369573338008, -980.8949562287198, -984.2158239105938, -977.4496625118336, -980.726601044199, -973.8811045539642, -976.9319797863454, -970.1568542610194, -973.1378281462194, -966.2317771362859, -969.0344962614627, -962.0862458601505, -964.938267973138, -957.894231638059, -960.8432839451134, -953.6268001678945, -956.2382089215407, -948.849917425775, -951.5404603686347, -944.1756993905246, -946.7035527213593, -939.1412110563824, -941.6328266048149, -933.9204958626533, -936.2116012459737, -928.582683739729, -930.7138520302324, -922.792432999785, -924.861270829646, -916.9220283412242, -918.6501396710146, -910.6287633592647, -912.2352070682673, -903.936090133996, -905.4786663052537, -897.4244876583743, -898.6675468484573, -890.2214712259138, -891.4202704777181, -883.0964014950787, -884.2213260239323, -875.5378908173325, -876.5560292539403, -866.7663383740919, -865.5463448288301, -861.0946339579541, -859.9192201425722, -863.4253116836862, -862.1750004915793, -870.4662969332085, -869.158108917617, -877.6025908875208, -875.7457802188519, -884.051159628285, -882.3039973245495, -890.5113019009541, -888.4722047626929, -896.4339521920137, -894.2918955779314, -902.3278707634663, -900.0244688465482, -907.7369117459075, -905.3557038852223, -913.1837702229413, -910.6472040857307, -918.2273714626044, -915.6715484664301, -923.0268334654884, -920.4405819355661, -927.7359324826439, -925.0419786824423, -932.3364866015299, -929.3518270011045, -936.437165966383, -933.6119047176289, -940.6622391542587, -937.7973020685804, -944.6954712045572, -941.7160613411952, -948.5418675816281, -945.438076684728, -952.292854262143, -948.9830678801509, -955.7688833051843, -952.4114068873832, -959.0583849553504, -955.6555390089115, -962.2932855967338, -958.8764899240323, -965.4761488422309, -962.0502216833202, -968.5242086947419, -964.9765085138506, -971.4238175173487, -967.8556146545297, -974.2583878901105, -970.7675058250807, -977.177551712417, -973.7142384301706, -979.9784672455198, -976.4226880917504, -982.7525537813372, -978.9731154937735, -996.3245605933862, -996.2980508169767, -996.4371730365256, -996.356985451599, -996.2640459209051, -996.2960990922329, -996.2927043018863, -996.2857962126509, -996.2411496337027, -996.3282979879568, -996.2551438051287, -996.270109442883, -996.1730407615469, -996.3111667639005, -996.2400292940056, -996.2614145848256, -996.2891713011195, -996.228854689427, -996.3386556966907, -996.2825677079745, -996.3093774381541, -996.3486287557898, -996.2465124530554, -996.3356221257545, -996.3475861701736, -996.2789541080983, -996.3117752705803, -996.281075314655, -996.3023719978992, -996.3265099086129, -996.2305273716393, -996.3285015081365, -996.4455813686363, -996.3202488959723, -996.312787015986, -996.2422906696247, -996.3233949062087, -996.3554728220297, -996.3182111227798, -996.3154862937881, -996.3417730377114, -996.2855326883491, -996.2890354978099, -996.3255867889948, -996.3967638309496, -996.2643703016547, -996.3577584321756, -996.2599907959866, -996.305830602596, -996.2722246850954, -996.3512908813591, -996.4252430873275, -996.2237747509171, -996.3264429544797, -996.2863873374208, -996.3355129990614, -996.2970515777597, -996.1957171069553, -996.2624608798778, -996.2549818664374, -996.2838298963125, -996.2246762685118, -996.2220371901858, -996.2011452670413, -996.2381663441756, -996.2126251946975, -996.2470320599987, -996.254178024341, -996.2380263059968, -996.1570818433684, -996.2196216361954, -996.3584104525471, -996.3688280378392, -996.3475770595142, -996.4046057239575, -996.339517691069, -996.3134648045307, -996.3353410365708, -996.3690404407007, -996.3140324454689, -996.3277601843238, -996.3370331499955, -996.360596327504, -996.3303781363466, -996.2903023025974, -996.3272820940383, -996.356530735955, -996.4032626110093, -996.23532396872, -996.2330888938486, -996.3304662657065, -996.31016980206, -996.412367709052, -996.3598996924284, -996.460692750421, -996.3713386465315, -996.4034794655108, -996.3688038929358, -996.3614245256631, -996.312001114291, -946.8094090644518, -946.2931786867666, -945.9753270801957, -944.9247749619426, -945.5671187056523, -944.4258927221344, -943.5756607789808, -944.1591646718425, -945.3989214241228, -946.4513020988943, -946.364829402426, -945.0394023331573, -945.5361227973244, -944.6015465812234, -947.5238622561719, -946.3184752055859, -944.1081976858059, -944.7608877506391, -943.4721551846433, -945.1302607323923, -943.3051584454734, -944.0124686437466, -945.0419674336281, -945.7515761513478, -945.848644006619, -946.1203559027599, -944.0825098311743, -944.1915652203843, -945.1545379190593, -943.7796687336067, -945.2985235077704, -944.593054132265, -942.4093736963387, -944.3693796270145, -944.7587442551594, -943.9593518093534, -944.3475032031583, -942.8768189681887, -942.8781921158916, -943.1426241192676, -944.0834541232744, -945.7198328537143, -942.7950151009409, -946.5241716040364, -944.1072279188957, -945.4859872543329, -945.4491182715865, -946.2014717610091, -943.811335319815, -945.1195756133002, -999.1375859414456, -997.0868915504179, -996.3787174784709, -992.707255109835, -996.3439347195563, -992.7186998726238, -999.0069636114995, -995.4609516344508, -998.243302245709, -998.1863726634738, -995.4557810575297, -998.9766823844848, -992.6681213814745, -996.1549974928976, -989.734606215241, -993.208159149297, -986.7480860799496, -990.1147879499158, -983.6411570406517, -987.0766647275495, -980.4763429528775, -983.721656308956, -977.0275998849083, -980.2150082111339, -973.4977063985662, -976.6553989088443, -969.8015450955791, -972.7992014352612, -965.9593409386998, -968.9604604613469, -961.8835810884157, -964.8543691325467, -957.7395577152847, -960.5360912898341, -953.3361621350059, -956.0497733420079, -948.7025421476192, -951.4301768544346, -943.9316666270051, -946.3943231549656, -938.9238141419273, -941.363590068785, -933.6844917757826, -936.098485120563, -928.2421355914712, -930.4870877782541, -922.5235448494186, -924.5542884949846, -916.5437989374659, -918.4345787686107, -910.3951382040987, -912.0933762564719, -903.7317171882241, -905.3004957135881, -897.0515994927282, -898.422626186335, -890.0041973521647, -891.3021285676214, -882.6210815828363, -883.9119613596476, -873.8441299555416, -872.627920179415, -867.9194072300552, -866.5632994652387, -870.0377405900726, -868.5876120443281, -876.9228856674563, -875.258362523723, -883.5858998410949, -881.6767514152061, -889.8998637098575, -887.9321425486378, -895.9333701894157, -893.822708265101, -901.8136207843136, -899.5294489418011, -907.3935986855486, -905.0686809034669, -912.6893912133128, -910.2358934537715, -917.7917945715972, -915.331254635319, -922.7153231360799, -920.106238826842, -927.4266523761689, -924.7355316361491, -931.8863381647079, -929.1610490810772, -936.1826854944611, -933.3431946982664, -940.3472745279269, -937.3517772267223, -944.3052822775371, -941.239824065442, -948.0640050724996, -944.8634462165328, -951.6349684351517, -948.4164993246604, -955.1079671382149, -951.846054930088, -958.462447752846, -955.0731491322831, -961.6799662981512, -958.233541044483, -964.6724978734073, -961.1952509421835, -967.6604980028651, -964.135479339714, -970.4811427428522, -967.0161177804412, -973.3081828774366, -969.7576563671037, -976.1263725608824, -972.4578690394183, -978.7898770902912, -975.1800623736772, -981.5536546330741, -977.865733423866, -984.1745552878638, -980.4236299594995, -990.4552965909488, -994.1555678832538, -998.8267495460004, -995.1531248383717, -996.4700921614431, -992.8343724161005, -999.2296332526466, -995.55892043934, -998.1083579147153, -998.3191244320788, -995.329211324778, -998.8087421945556, -992.4044401770043, -995.9768639185959, -989.518264172706, -993.0033391523039, -986.5082906790758, -989.8917548057007, -983.4051627087365, -986.727529548355, -980.0592429129028, -983.3899342398709, -976.6171428524813, -979.847482029053, -973.1415445593539, -976.251745326389, -969.3908666721991, -972.469666746636, -965.5646452780766, -968.5183413532532, -961.4427749612332, -964.4414492610131, -957.3245720610676, -960.1177799335455, -952.8077210929268, -955.6743881994198, -948.2931289755916, -950.9285542835605, -943.4339892442904, -946.0489259178521, -938.4146361132143, -940.9441895959244, -933.2469395299377, -935.5146600113785, -927.6794463011274, -929.8623027230578, -922.053266665047, -924.0805874487951, -916.0170588278179, -917.8844952662203, -909.6999042873713, -911.5386086095232, -903.1708421696758, -904.7951052027202, -896.3415603301246, -897.9044413111114, -889.4288715897737, -890.7527357551526, -882.1127114829033, -883.4174003765047, -873.400679253602, -872.1749553897271, -867.6127054646868, -866.1956889015328, -869.7632344555032, -868.1401851404871, -876.4918102443817, -874.9411422658377, -883.1554612850059, -881.3402701516152, -889.5947602070219, -887.6210399173842, -895.6903365332973, -893.5593450973629, -901.6234755989071, -899.3056939087401, -907.158054272717, -904.8507250992116, -912.5171098922392, -910.1097932986186, -917.779921763843, -915.1655057735034, -922.5805947013496, -919.917073020808, -927.2785992044091, -924.4970888427515, -931.8017085949468, -929.036196610753, -936.2022349357776, -933.271426542221, -940.2859180078367, -937.2534058835527, -944.1453579871732, -941.0405634351864, -948.01002129682, -944.8027722508205, -951.5628629699777, -948.2625094615923, -955.0151413029125, -951.6987600829634, -958.3242114126851, -954.9814099072255, -961.5332823662939, -958.056368130512, -964.7041121255033, -961.1751040460622, -967.714720072775, -964.0706195424145, -970.5840235910273, -966.9839604848494, -973.3505593967475, -969.7274608012049, -976.1180351405992, -972.4801163575812, -978.8187987911306, -975.16991903301, -981.4787465685195, -977.8052005010195, -984.1720586965812, -980.3931363029214, -990.3857999994661, -994.1695957426937, -998.8179367490438, -995.1683514595434, -996.4948820109566, -992.8610684711675, -999.1577618241072, -995.546838886492, -998.0641042077923, -998.3532400438999, -995.2790068175618, -998.8988116732344, -992.4354564621208, -996.0099097611092, -989.5619009257834, -992.9819862356171, -986.4809127326535, -989.9871892046131, -983.4062261014406, -986.7429508184077, -980.0078376154725, 